vi "HeartBeatDetectOffline2.vi"() -> ()   [LabVIEW 2014, in "Phonocardiography.lvlib"]
uses:
  <vilib>/Waveform/WDTOps.llb/WDT Index Channel DBL.vi
  <vilib>/Waveform/WDTOps.llb/WDT Get Waveform Time Array DBL.vi
  Phonocardiography.lvlib
panel:
  in  "Remove\nEctopic Beats":bool=TRUE
  out "pNN50 [%]":dbl=10.344827586206897 format="%0.2f"
  out "rMSSD  [ms]":dbl=56.69079988743271 format="%0.2f"
  out "sdRR [ms]":dbl=155.73913956064249 format="%0.2f"
  out "Mean RR [ms]":dbl=679.0314769975785 format="%0.2f"
  out "Mean heart rate [BPM]":dbl=88.36114676936246
  in  "Negate":bool
  out "Heart rate":cluster{"HR X":dbl[], "HR":dbl[]}(graph)={"HR X"=[0.9536507936507932, 1.7804988662131511, 2.524807256235827, 3.2744671201814044, 4.085170068027209, 4.935691609977322, 5.717823129251698, 6.664217687074827, 7.49442176870748, 8.24662131519274, 8.931065759637184, 9.6128798185941, 10.405986394557818, 11.348027210884348, 12.258866213151922, 13.136780045351468, 13.961088435374144, 14.727165532879813, 15.434376417233553, 16.08961451247165, 16.721904761904756, 17.338321995464845, 17.933514739229018, 18.513469387755094, 19.077641723356003, 19.63292517006802, 20.182403628117907, 20.724172335600898, 21.26467120181405, 21.80018140589568, 22.325532879818585, 22.852698412698402, 23.38702947845804, 23.93859410430838, 24.48843537414965, 25.032743764172324, 25.566167800453503, 26.094965986394545, 26.626666666666654, 27.148843537414955, 27.667120181405885, 28.183219954648514, 28.69315192743763, 29.19600907029477, 29.70113378684806, 30.20426303854874, 30.718911564625838, 31.25142857142856, 31.85287981859409, 32.489795918367335, 33.11401360544216, 33.734331065759626, 34.587845804988646, 35.485986394557806, 36.427664399092954, 37.37106575963717, 38.321088435374136, 39.26984126984125, 40.178049886621295], "HR"=[71.55993076590225, 72.56472136902153, 80.61174750182794, 80.03629764065343, 74.00984560304319, 70.54495041057912, 76.71344079786621, 63.39850488786662, 72.27138643067849, 79.76606776799711, 87.66233766233783, 88.0005321271783, 75.65187557182081, 63.69150779896015, 65.87333200557657, 68.34383717326173, 72.78829225352112, 78.32109874496807, 84.84032320123139, 91.56976744186045, 94.89312867594295, 97.33666862860537, 100.80768058518736, 103.45636534250875, 106.35048231511234, 108.05292388108468, 109.19445361505448, 110.74836765444552, 111.00855848296688, 112.04268292682941, 114.20925414364623, 113.81624225739887, 112.28993379731786, 108.78145041933905, 109.12240184757502, 110.2316280619899, 112.48087060023806, 113.4648370497429, 112.84544524053209, 114.90359562271999, 115.76828841442064, 116.25659050966627, 117.6627534685167, 119.31818181818207, 118.78254623810332, 119.25365062195846, 116.58442016214268, 112.67245784363834, 99.75870909365125, 94.20393050412952, 96.12031386225006, 96.72466734902676, 70.29755579171136, 66.80468592203607, 63.716047004430656, 63.599653879434875, 63.15638724460529, 63.240917782027125, 66.06411664835723]}
  out "Heart beats":cluster{"Peaks X":dbl[], "Peaks Y":dbl[]}[](graph)=[{"Peaks X"=array[450560 elements], "Peaks Y"=array[450560 elements]}, {"Peaks X"=[0.11519274376417228, 0.9536507936507932, 1.7804988662131511, 2.524807256235827, 3.2744671201814044, 4.085170068027209, 4.935691609977322, 5.717823129251698, 6.664217687074827, 7.49442176870748, 8.24662131519274, 8.931065759637184, 9.6128798185941, 10.405986394557818, 11.348027210884348, 12.258866213151922, 13.136780045351468, 13.961088435374144, 14.727165532879813, 15.434376417233553, 16.08961451247165, 16.721904761904756, 17.338321995464845, 17.933514739229018, 18.513469387755094, 19.077641723356003, 19.63292517006802, 20.182403628117907, 20.724172335600898, 21.26467120181405, 21.80018140589568, 22.325532879818585, 22.852698412698402, 23.38702947845804, 23.93859410430838, 24.48843537414965, 25.032743764172324, 25.566167800453503, 26.094965986394545, 26.626666666666654, 27.148843537414955, 27.667120181405885, 28.183219954648514, 28.69315192743763, 29.19600907029477, 29.70113378684806, 30.20426303854874, 30.718911564625838, 31.25142857142856, 31.85287981859409, 32.489795918367335, 33.11401360544216, 33.734331065759626, 34.587845804988646, 35.485986394557806, 36.427664399092954, 37.37106575963717, 38.321088435374136, 39.26984126984125, 40.178049886621295], "Peaks Y"=[0.26409912109375, 0.216064453125, 0.231689453125, 0.2972412109375, 0.2186279296875, 0.310516357421875, 0.252410888671875, 0.3045654296875, 0.187164306640625, 0.24078369140625, 0.215057373046875, 0.3526611328125, 0.2615966796875, 0.229461669921875, 0.192779541015625, 0.189361572265625, 0.17205810546875, 0.186737060546875, 0.212005615234375, 0.185272216796875, 0.16400146484375, 0.175933837890625, 0.1873779296875, 0.1800537109375, 0.20709228515625, 0.20452880859375, 0.2001953125, 0.218231201171875, 0.222015380859375, 0.217681884765625, 0.201202392578125, 0.212066650390625, 0.219879150390625, 0.2449951171875, 0.2816162109375, 0.262664794921875, 0.234039306640625, 0.287567138671875, 0.267730712890625, 0.258544921875, 0.271209716796875, 0.25408935546875, 0.272186279296875, 0.230987548828125, 0.265380859375, 0.269317626953125, 0.267486572265625, 0.289703369140625, 0.216644287109375, 0.20257568359375, 0.270477294921875, 0.246978759765625, 0.403839111328125, 0.436309814453125, 0.427947998046875, 0.40887451171875, 0.40252685546875, 0.448974609375, 0.42376708984375, 0.371551513671875]}]
  in  "Max time to peak\nfrom threshold (ms)":dbl=150.0
  in  "Threshold mult":dbl=0.35 min=-1.0 max=1.0 step=0.05
  in  "Min time between\nbeats (ms)":dbl=400.0
  in  "width (threshold)":i32=3
  in  "File Path Control":path=path "C:/Users/Tamas/Documents/Projektek/Magzati szívhang/Felvételek cikkhez/valsalva5.wav"
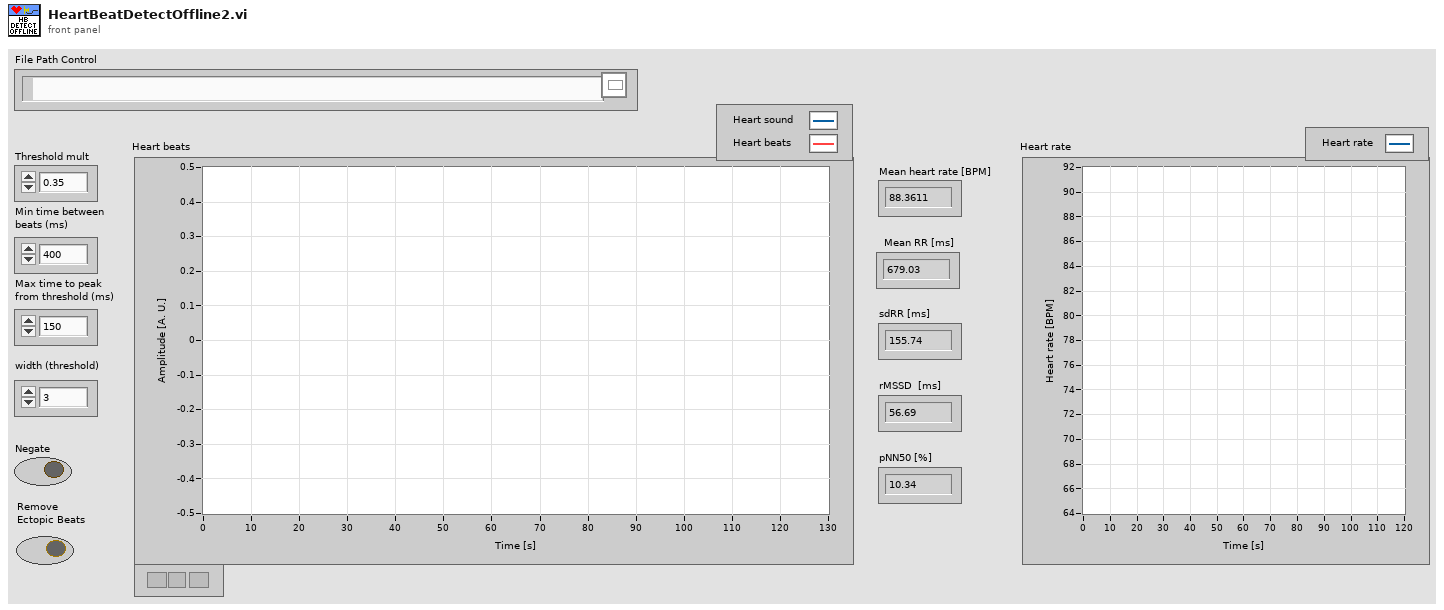
[diagram p1: front panel]
types:
  T1 = typedef "LVCursorListTypeDef.ctl" = cluster{"Name":string, "Color":u32, "Style":u8, "Point Style":u8, "Name Visible":bool, "Allow Drag":bool, "Cursor Mode":u32, "Plot":i32, "Index":i32, "Position":cluster{"X":dbl, "Y":dbl}, "X Scale":u32, "Y Scale":u32, "Watch Plots":i32[], "Watch All Plots":bool, "Plot Area":i32, "Label Offset":cluster{"X":dbl, "Y":dbl}}[]
  T2 = cluster{"Name":string, "Color":u32, "Style":u8, "Point Style":u8, "Name Visible":bool, "Allow Drag":bool, "Cursor Mode":u32, "Plot":i32, "Index":i32, "Position":cluster{"X":dbl, "Y":dbl}, "X Scale":u32, "Y Scale":u32, "Watch Plots":i32[], "Watch All Plots":bool, "Plot Area":i32, "Label Offset":cluster{"X":dbl, "Y":dbl}}
  T3 = cluster{"Name":string, "Color":u32, "Style":u8, "Point Style":u8, "Name Visible":bool, "Allow Drag":bool, "Cursor Mode":u32, "Plot":i32, "Index":i32, "Position":cluster{"X":dbl, "Y":dbl}, "X Scale":u32, "Y Scale":u32, "Watch Plots":i32[], "Watch All Plots":bool, "Plot Area":i32, "Label Offset":cluster{"X":dbl, "Y":dbl}}[]
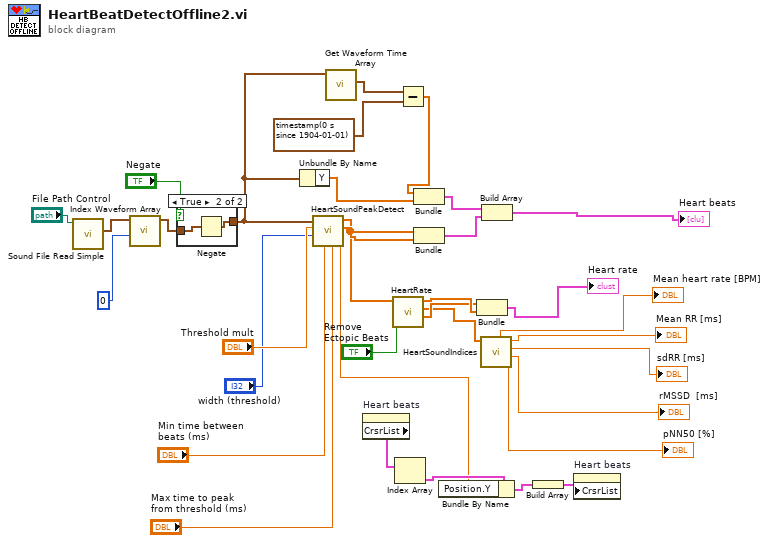
[diagram p0: block diagram]
diagram:
  n1 = call <vilib>:"Sound File Read Simple.vi"("path"="File Path Control") -> ("data"=w33:waveform(dbl)[])  [unwired: 7 in, 3 out]
  n2 = call-poly <vilib>:"Index Waveform Array.vi"("index"=0, "waveform array"=w33) -> ("waveform"=w11:waveform(dbl))  [unwired: 8 in, 1 out]
  n3 = case shown="True" "Negate" {
    tunnel: w11 -> [w35 w37]
    tunnel: [w35 w36] -> w10
    frame False {
    }
    frame True {
      n4 = Negate(x=w37) -> (-x=w36:waveform(dbl))
    }
  }
  n5 = Unbundle By Name(w10) -> ("Y"=w19:dbl[])
  n6 = call "HeartSoundPeakDetect.vi"("Max time to peak\nfrom threshold (ms)"="Max time to peak\nfrom threshold (ms)", "Min time between\nbeats (ms)"="Min time between\nbeats (ms)", "width (threshold)"="width (threshold)", "Threshold multiplier"="Threshold mult", "Sound"=w10) -> ("Threshold"=w12:dbl, "Peaks Y"=w27:dbl[], "Peaks X"=w24:dbl[])  [unwired: 4 in]
  n7 = call-poly <vilib>:"Get Waveform Time Array.vi"("waveform in"=w10) -> ("X array"=w22:timestamp[])  [unwired: 9 in, 1 out]
  n8 = property on="Heart beats" class="XYGraph (strict)"() -> ("CrsrList"=w14:T1)  [unwired: 2 in, 2 out]
  n9 = call "HeartRate.vi"("Remove Ectopic?"="Remove\nEctopic Beats", "Peaks X in"=w24) -> ("X [s]"=w8:dbl[], "RR intervals [ms]"=w7:dbl[], "Heart Rate [BPM]"=w23:dbl[])  [unwired: 7 in]
  n10 = Index Array(array=w14) -> (element=w16:T2)  [unwired: 1 in]
  n11 = Subtract(x=w22, y=timestamp(0 s since 1904-01-01) ("Xo")) -> (x-y=w20:dbl[])
  n12 = Bundle(w20, "Y"=w19) -> (w26:cluster{dbl[], "Y":dbl[]})  [unwired: 1 in]
  n13 = Bundle("Peaks X"=w24, "Peaks Y"=w27) -> (w25:cluster{"Peaks X":dbl[], "Peaks Y":dbl[]})  [unwired: 1 in]
  n14 = Bundle By Name(cluster=w16, "Position.Y"=w12) -> (w15:T2)
  n15 = Bundle("X [s]"=w8, "Heart Rate [BPM]"=w23) -> (→"Heart rate":cluster{"X [s]":dbl[], "Heart Rate [BPM]":dbl[]})  [unwired: 1 in]
  n16 = call "HeartSoundIndices.vi"("RR intervals [ms]"=w7) -> ("pNN50 [%]"=→"pNN50 [%]":dbl, "rMSSD  [ms]"=→"rMSSD  [ms]":dbl, "sdRR [ms]"=→"sdRR [ms]":dbl, "Mean RR [ms]"=→"Mean RR [ms]":dbl, "Mean heart rate [BPM]"=→"Mean heart rate [BPM]":dbl)  [unwired: 6 in]
  n17 = Build Array(w26, w25) -> (→"Heart beats":cluster{"Peaks X":dbl[], "Peaks Y":dbl[]}[])
  n18 = Build Array(w15) -> (w13:T3)
  n19 = property on="Heart beats" class="XYGraph (strict)"("CrsrList"=w13) -> ()  [unwired: 2 in, 2 out]
